vi "Controle_Manip_Main_GUI_Backup2.vi"() -> ()   [LabVIEW 2019] (continued)
                                n1251 = local write "PH_Settings_Params"(w1611) -> ()
                                }
                                frame #2 {
                                n1252 = local read "Spectrum End Wavelength (nm)"() -> (w1629:dbl)
                                n1253 = local read "Spectrum Step Wavelength (nm)"() -> (w1627:dbl)
                                n1254 = local read "Spectrum Start Wavelength (nm)"() -> (w1626:dbl)
                                n1255 = Subtract(x=w1629, y=w1626) -> (x-y=w1631:dbl)
                                n1256 = Divide(x=w1631, y=w1627) -> (x/y=w1630:dbl)
                                n1257 = Increment(x=w1630) -> (x+1=w1628:dbl)
                                n1258 = for {
                                N: w1628 -> [_]
                                tunnel: w1627 -> [w1634]
                                tunnel: w1626 -> [w1635]
                                shift-right: [w1636] -> w1622
                                shift-left: dbl[] [] -> [w1638]
                                shift-right: [w1639] -> w1623
                                shift-left: dbl[] [] -> [w1640]
                                i -> [w1644]
                                stop <- w1632 stop-if-true
                                n1259 = Multiply(x=w1644, y=w1634) -> (x*y=w1643:dbl)
                                n1260 = Add(x=w1635, y=w1643) -> (x+y=w1633:dbl)
                                n1261 = local read "ESP300 COM Port"() -> (w1642:refnum<visa-resource-name>)
                                n1262 = stacked-sequence {
                                tunnel: w1633 -> [w1647 _ w1654 _]
                                tunnel: w1642 -> [w1652 _ _ _]
                                tunnel: [_ _ w1661 _] -> w1641
                                tunnel: w1640 -> [w1650 _ _ _]
                                tunnel: [w1649 _ _ _] -> w1639
                                tunnel: [_ _ _ w1679] -> w1632
                                frame #0 {
                                w1645 = u16 1 items=["Detection"=1, "Excitation"=2] ("HR mode")
                                n1263 = call "MotorWL2Pos.vi"("Mono2 Center WL"=w1647, "HR mode"=w1645) -> ("Mono2 Position"=w1648:dbl)
                                n1264 = control-ref of="Mono2 Wavelength (nm)"() -> (w1646:refnum<vi>)
                                n1265 = control-ref of="Mono2 Motor Pos"() -> (w1651:refnum<vi>)
                                n1266 = call "subVI_Mono2Go2Posv2.vi"("Mono2 Motor Pos"=w1651, "Mono2 Wavelength (nm)"=w1646, "HR mode"=w1645, "Postion (Unit)"=w1648, "ESP300 COM Port"=w1652) -> ()  [unwired: 2 out]
                                n1267 = Insert Into Array(array=w1650, new element=w1647) -> (w1649:dbl[])  [unwired: 1 in]
                                }
                                frame #1 {
                                n1268 = Wait (ms)(milliseconds to wait=u32 20) -> ()  [unwired: 1 out]
                                }
                                frame #2 {
                                n1269 = local read "Photodiode error out"() -> (w1655:errorcluster)
                                n1270 = local read "Photodiode handle out"() -> (w1658:refnum<visa-resource-name>)
                                n1271 = Tick Count (ms)() -> (millisecond timer value=w1664:u32)
                                n1272 = call <instrlib>:"TLPM Set Wavelength.vi"("error in (no error)"=w1655, "Wavelength (0.0)"=w1654, "instrument handle"=w1658) -> ("error out"=w1656:errorcluster, "instrument handle out"=w1657:refnum<visa-resource-name>)  [unwired: 7 in]
                                n1273 = while {
                                shift-right: [w1674] -> w1659
                                shift-left: w1657 -> [w1677]
                                shift-right: [w1675] -> w1660
                                shift-left: w1656 -> [w1676]
                                tunnel: w1664 -> [w1672]
                                shift-right: [w1666] -> w1663
                                shift-left: dbl[] [] -> [w1667]
                                stop <- w1669 stop-if-true
                                n1274 = Tick Count (ms)() -> (millisecond timer value=w1673:u32)
                                n1275 = control-ref of="Excitation Power (uW)"() -> (w1665:refnum<vi>)
                                n1276 = local read "Acq Time (ms)"() -> (w1670:dbl)
                                n1277 = Subtract(x=w1673, y=w1672) -> (x-y=w1671:u32)
                                n1278 = call <instrlib>:"TLPM Measure Power.vi"("error in (no error)"=w1676, "instrument handle"=w1677) -> ("error out"=w1675:errorcluster, "Power"=w1668:dbl, "instrument handle out"=w1674:refnum<visa-resource-name>)  [unwired: 7 in]
                                n1279 = property class="DigNum (strict)"(reference=w1665, "Value"=w1668) -> ()  [unwired: 1 in, 2 out]
                                n1280 = Insert Into Array(array=w1667, new element=w1668) -> (w1666:dbl[])  [unwired: 1 in]
                                n1281 = Greater?(x=w1671, y=w1670) -> (0:w1669:bool)
                                }
                                n1282 = local write "Photodiode handle out"(w1659) -> ()
                                n1283 = local write "Photodiode error out"(w1660) -> ()
                                n1284 = call-poly <vilib>:"Mean.vi"("X"=w1663) -> ("mean"=w1661:dbl)  [unwired: 1 out]
                                }
                                frame #3 {
                                n1285 = control-ref of="MasterStop"() -> (w1678:refnum<vi>)
                                n1286 = control-ref of="Stop Spectrum Custom"() -> ()  [unwired: 1 out]
                                n1287 = property class="Bool (strict)"(reference=w1678) -> ("Value"=w1679:bool)  [unwired: 1 in, 2 out]
                                }
                                }
                                n1288 = Insert Into Array(array=w1638, new element=w1641) -> (w1636:dbl[])  [unwired: 1 in]
                                n1289 = Bundle(w1639, w1636) -> (w1637:cluster{dbl[], dbl[]})  [unwired: 1 in]
                                n1290 = property on="CCD 1D Spectrum Main" class="XYGraph (strict)"("Value"=w1637) -> ()  [unwired: 2 in, 2 out]
                                }
                                n1291 = local write "Data PL Custom Diode Spectrum"(w1622) -> ()
                                n1292 = local write "Wavelength calibration"(w1623) -> ()
                                }
                                frame #3 {
                                n1293 = property on="Elapsed (s)" class="DigNum (strict)"("Visible"=FALSE) -> ()  [unwired: 2 in, 2 out]
                                n1294 = control-ref of="Shutter Ctrls"() -> (w1682:refnum<vi>)
                                n1295 = local read "KCube Shutter On?"() -> (w1681:bool)
                                n1296 = control-ref of="KCube Shutter Device Reference"() -> (w1683:refnum<vi>)
                                n1297 = call "Shutter.vi"("KCube Shutter Device Reference 2"=w1683, "Shutter Ctrls 2"=w1682, "Shutter on?"=w1681) -> ()
                                }
                                }
                              }
                            }
                          }
                          frame #3 {
                            n1298 = property on="Save Custom Diode Spectrum" class="Bool (strict)"("Visible"=TRUE) -> ()  [unwired: 2 in, 2 out]
                            n1299 = control-ref of="MasterPause"() -> (w1685:refnum<vi>)
                            n1300 = control-ref of="MasterStop"() -> (w1687:refnum<vi>)
                            n1301 = local read "Scan Spectrum Cust Params"() -> (w1691:refnum<vi>[])
                            n1302 = property on="Acquire Custom Diode Spectrum" class="Bool (strict)"("Value"=FALSE ("Acquire Custom Diode Spectrum")) -> ()  [unwired: 2 in, 2 out]
                            n1303 = control-ref of="ExperimentStopped?"() -> (w1686:refnum<vi>)
                            n1304 = call "CheckStopAndReset.vi"("ExperimentStopped?"=w1686, "MasterStop"=w1687, "MasterPause"=w1685) -> ()
                            n1305 = call "Enable&Disable_Controls.vi"("Enum"=enum16{"Enabled", "Disabled", "Disabled&Grayed"}."Enabled", "References"=w1691) -> ()  [unwired: 1 in]
                            n1306 = local write "Background taken?"(FALSE ("Background taken?")) -> ()
                          }
                        }
                      }
                      frame "Acquire PLE" {
                        n1307 = stacked-sequence {
                          frame #0 {
                            # "background"
                            n1308 = local read "Background taken?"() -> (w1692:bool)
                            n1309 = case shown="False" w1692 {
                              frame False {
                                n1310 = stacked-sequence {
                                tunnel: [_ _ w1738] -> w1693
                                frame #0 {
                                n1311 = property on="CCD 1D Spectrum Main" class="XYGraph (strict)"("YScale.Offset"=0.0 ("Y Scale.Offset and Multiplier:Offset")) -> ()  [unwired: 2 in, 2 out]
                                }
                                frame #1 {
                                # "make sure shutter is closed"
                                n1312 = local read "KCube Shutter On?"() -> (w1724:bool)
                                n1313 = control-ref of="Shutter Ctrls"() -> (w1728:refnum<vi>)
                                n1314 = property class="Ring (strict)"(reference=w1728) -> ("Value"=w1727:u16)  [unwired: 1 in, 2 out]
                                n1315 = control-ref of="KCube Shutter Device Reference"() -> (w1729:refnum<vi>)
                                n1316 = Equal?(x=w1727, y=u16 0) -> (x = y?=w1725:bool)
                                n1317 = case shown="False" w1725 {
                                tunnel: w1729 -> [w1732 _]
                                tunnel: w1728 -> [w1731 _]
                                tunnel: w1724 -> [w1730 _]
                                frame False {
                                n1318 = call "Shutter.vi"("KCube Shutter Device Reference 2"=w1732, "Shutter Ctrls 2"=w1731, "Shutter on?"=w1730) -> ()
                                }
                                frame True {
                                }
                                }
                                }
                                frame #2 {
                                # "acquire"
                                n1319 = local read "LightField Automation error out"() -> (w1736:errorcluster)
                                n1320 = local read "LightField Automation out"() -> (w1737:refnum<class "LightField Automation.lvclass">)
                                n1321 = local read "Accumulations"() -> (w1733:dbl)
                                n1322 = call "LFA_Capture.vi"("error in (no error)"=w1736, "Frames"=w1733, "LightField Automation in"=w1737) -> ("error out"=w1735:errorcluster, "Data"=w1738:T26, "LightField Automation out"=w1734:refnum<class "LightField Automation.lvclass">)  [unwired: 6 in]
                                n1323 = local write "LightField Automation error out"(w1735) -> ()
                                n1324 = local write "LightField Automation out"(w1734) -> ()
                                }
                                }
                                n1325 = local read "Acq Mode"() -> (w1694:T3)
                                n1326 = case shown="\"Spectrum\", Default" w1694 {
                                selector: w1694 -> [w1695 w1713]
                                tunnel: w1693 -> [w1696 w1714]
                                frame "Spectrum", Default {
                                n1327 = stacked-sequence {
                                tunnel: w1696 -> [_ w1707 _ _]
                                tunnel: w1695 -> [_ w1705 _ _]
                                frame #0 {
                                n1328 = property on="CCD 2D Image Main" class="IntGraph (strict)"("Visible"=FALSE) -> ()  [unwired: 2 in, 2 out]
                                n1329 = property on="CCD 1D Spectrum Main" class="XYGraph (strict)"("Visible"=TRUE) -> ()  [unwired: 2 in, 2 out]
                                }
                                frame #1 {
                                n1330 = local read "Wavelength calibration"() -> (w1704:dbl[])
                                n1331 = local read "CCD ROI"() -> (w1700:T20)
                                n1332 = Divide(x=1239.842, y=w1704) -> (x/y=w1702:dbl[])
                                n1333 = call "PrepareData4Graph.vi"("Wavelength nm"=w1702, "DataLF"=w1707, "CCD ROI"=w1700, "AcqMode"=w1705, "Data type"=T30."Spectre") -> ("Spectrum"=w1706:cluster{"Array 2":dbl[], "Array":dbl[]}, "PLInt out"=w1699:dbl[])  [unwired: 2 in, 2 out]
                                n1334 = local write "CCD 1D Spectrum Main"(w1706) -> ()
                                n1335 = local write "BackgroundSpec"(w1699) -> ()
                                }
                                frame #2 {
                                n1336 = local read "BackgroundSpec"() -> (w1708:dbl[])
                                n1337 = call-poly <vilib>:"Mean.vi"("X"=w1708) -> ("mean"=w1710:dbl)  [unwired: 1 out]
                                n1338 = Negate(x=w1710) -> (-x=w1709:dbl)
                                n1339 = property on="CCD 1D Spectrum Main" class="XYGraph (strict)"("YScale.Offset"=w1709) -> ()  [unwired: 2 in, 2 out]
                                }
                                frame #3 {
                                n1340 = local write "Background taken?"(TRUE ("Background taken?")) -> ()
                                n1341 = property on="Background substract" class="Enum (strict)"("Value"=enum16{"None", "Shutter"}."None" ("Background substract")) -> ()  [unwired: 2 in, 2 out]
                                }
                                }
                                }
                                frame "Image" {
                                n1342 = stacked-sequence {
                                tunnel: w1714 -> [_ w1722]
                                tunnel: w1713 -> [_ w1720]
                                frame #0 {
                                n1343 = property on="CCD 1D Spectrum Main" class="XYGraph (strict)"("Visible"=FALSE) -> ()  [unwired: 2 in, 2 out]
                                n1344 = property on="CCD 2D Image Main" class="IntGraph (strict)"("Visible"=TRUE) -> ()  [unwired: 2 in, 2 out]
                                }
                                frame #1 {
                                n1345 = local read "Wavelength calibration"() -> (w1721:dbl[])
                                n1346 = local read "CCD ROI"() -> (w1717:T20)
                                n1347 = call "PrepareData4Graph.vi"("Wavelength nm"=w1721, "DataLF"=w1722, "CCD ROI"=w1717, "AcqMode"=w1720, "Data type"=T30."Spectre") -> ("Intensity Graph"=w1719:dbl[][])  [unwired: 2 in, 3 out]
                                n1348 = local write "CCD 2D Image Main"(w1719) -> ()
                                }
                                }
                                }
                                }
                              }
                              frame True {
                              }
                            }
                          }
                          frame #1 {
                            # "prep"
                            n1349 = control-ref of="MasterStop"() -> (w1758:refnum<vi>)
                            n1350 = control-ref of="MasterPause"() -> (w1755:refnum<vi>)
                            n1351 = local read "Spectrum Custom Mode"() -> (w1762:u16)
                            n1352 = local read "KCube Shutter On?"() -> (w1761:bool)
                            n1353 = local read "PLE Step (nm)"() -> (w1740:dbl)
                            n1354 = local read "PLE End (nm)"() -> (w1749:dbl)
                            n1355 = local read "Acq Time (ms)"() -> (w1760:dbl)
                            n1356 = local read "PLE Start (nm)"() -> (w1748:dbl)
                            n1357 = property class="Bool (strict)"(reference=w1758, "Visible"=TRUE) -> ()  [unwired: 1 in, 2 out]
                            n1358 = property class="Bool (strict)"(reference=w1755, "Visible"=TRUE) -> ()  [unwired: 1 in, 2 out]
                            n1359 = Bundle("Acq Time (ms)"=w1760, "PLE Start (nm)"=w1748, "PLE Step (nm)"=w1740, "PLE End (nm)"=w1749, "Spectrum Custom Mode"=w1762, "KCube Shutter On?"=w1761) -> (→"Scan PLE":T34)  [unwired: 1 in]
                            n1360 = control-ref of="PLE # Pts"() -> (w1746:refnum<vi>)
                            n1361 = Max & Min(x=w1748, y=w1749) -> (max(x,y)=w1744:dbl, min(x,y)=w1739:dbl)
                            n1362 = local read "Scan PLE AllParams"() -> (w1747:refnum<vi>[])
                            n1363 = property on="Experiment Graph Controls" class="TabCtl (strict)"("Value"=T25."PLE" ("Experiment Graph Controls")) -> ()  [unwired: 2 in, 2 out]
                            n1364 = Build Array (concatenate)(w1747, w1746) -> (w1745:refnum<vi>[])
                            n1365 = control-ref of="Elapsed (s)"() -> (w1753:refnum<vi>)
                            n1366 = property class="DigNum (strict)"(reference=w1753, "Visible"=TRUE) -> ()  [unwired: 1 in, 2 out]
                            n1367 = call "Enable&Disable_Controls.vi"("Enum"=enum16{"Enabled", "Disabled", "Disabled&Grayed"}."Disabled&Grayed", "References"=w1745) -> ()  [unwired: 1 in]
                            n1368 = Add(x=w1744, y=w1740) -> (x+y=w1741:dbl)
                            n1369 = Add(x=w1744, y=w1740) -> (x+y=w1743:dbl)
                            n1370 = property on="PLE Normalised Intensity" class="IntGraph (strict)"("XScale.Multiplier"=w1740, "XScale.Offset"=w1739, "YScale.Maximum"=1340.0 ("Y Scale.Range:Maximum"), "XScale.Minimum"=w1739, "XScale.Maximum"=w1743) -> ()  [unwired: 2 in, 2 out]
                            n1371 = property on="PLE Raw Intensity" class="IntGraph (strict)"("XScale.Multiplier"=w1740, "XScale.Offset"=w1739, "YScale.Maximum"=1340.0 ("Y Scale.Range:Maximum"), "XScale.Minimum"=w1739, "XScale.Maximum"=w1743) -> ()  [unwired: 2 in, 2 out]
                            n1372 = property on="PLE Laser Excitation Power" class="WFGraph (strict)"("XScale.Multiplier"=w1740, "XScale.Offset"=w1739, "XScale.Minimum"=w1739, "XScale.Maximum"=w1741) -> ()  [unwired: 2 in, 2 out]
                            n1373 = property on="PLE Integrated emission efficiency" class="WFGraph (strict)"("XScale.Multiplier"=w1740, "XScale.Offset"=w1739, "XScale.Minimum"=w1739, "XScale.Maximum"=w1741) -> ()  [unwired: 2 in, 2 out]
                          }
                          frame #2 {
                            n1374 = local read "Scan PLE"() -> (w1782:T1)
                            n1375 = Unbundle By Name(w1782) -> ("Acq Time (ms)"=w1775:dbl, "PLE start (nm)"=w1776:dbl, "PLE step (nm)"=w1777:dbl, "PLE end (nm)"=w1781:dbl)  [unwired: 2 out]
                            n1376 = Subtract(x=w1781, y=w1776) -> (x-y=w1780:dbl)
                            n1377 = Get Date/Time In Seconds() -> (seconds since 1Jan1904=w1771:timestamp)
                            n1378 = Divide(x=w1780, y=w1777) -> (x/y=w1779:dbl)
                            n1379 = Increment(x=w1779) -> (x+1=w1778:dbl)
                            n1380 = for {
                              N: w1778 -> [w1788]
                              tunnel: w1777 -> [w1804]
                              tunnel: w1776 -> [w1802]
                              tunnel: w1775 -> [w1800]
                              shift-right: [w1798] -> w1764
                              shift-left: dbl[] [] -> [w1799]
                              shift-right: [w1796] -> w1768
                              shift-left: i32[][] [] -> [w1797]
                              shift-right: [w1794] -> w1767
                              shift-left: dbl[][] [] -> [w1795]
                              tunnel: w1771 -> [w1790]
                              shift-right: [w1786] -> w1769
                              shift-left: dbl[] [] -> [w1787]
                              shift-right: [w1784] -> w1765
                              shift-left: dbl[] [] -> [w1785]
                              i -> [w1793]
                              stop <- w1805 stop-if-true
                              n1381 = Multiply(x=w1793, y=w1804) -> (x*y=w1803:dbl)
                              n1382 = Add(x=w1802, y=w1803) -> (x+y=w1801:dbl)
                              n1383 = Increment(x=w1793) -> (x+1=w1789:i32)
                              n1384 = Divide(x=w1789, y=w1788) -> (x/y=w1783:dbl)
                              n1385 = stacked-sequence {
                                tunnel: w1801 -> [_ w1819 _ _ w1831 _ _ _]
                                tunnel: w1800 -> [_ _ _ _ _ _ _ _]
                                tunnel: w1799 -> [_ _ _ _ w1828 _ _ _]
                                tunnel: [_ _ _ _ w1827 _ _ _] -> w1798
                                tunnel: w1797 -> [_ _ _ _ _ w1861 _ _]
                                tunnel: [_ _ _ _ _ w1860 _ _] -> w1796
                                tunnel: w1795 -> [_ _ _ _ _ w1859 _ _]
                                tunnel: [_ _ _ _ _ w1858 _ _] -> w1794
                                tunnel: w1790 -> [w1812 _ _ _ _ _ _ _]
                                tunnel: w1789 -> [w1811 _ _ _ _ _ _ _]
                                tunnel: w1788 -> [w1810 _ _ _ _ _ _ _]
                                tunnel: w1787 -> [_ _ _ _ _ w1857 _ _]
                                tunnel: [_ _ _ _ _ w1856 _ _] -> w1786
                                tunnel: w1785 -> [_ w1818 _ _ _ _ _ _]
                                tunnel: [_ w1817 _ _ _ _ _ _] -> w1784
                                tunnel: w1783 -> [_ _ w1824 _ _ _ _ _]
                                frame #0 {
                                # "prep"
                                n1386 = control-ref of="Expected (s)"() -> (w1808:refnum<vi>)
                                n1387 = call "Expectedtime.vi"("N"=w1810, "I"=w1811, "Reference time"=w1812) -> ("Expected time"=w1807:dbl, "Elapsed time"=w1809:dbl)
                                n1388 = property on="Elapsed (s)" class="DigNum (strict)"("Value"=w1809) -> ()  [unwired: 2 in, 2 out]
                                n1389 = property class="DigNum (strict)"(reference=w1808, "Value"=w1807) -> ()  [unwired: 1 in, 2 out]
                                }
                                frame #1 {
                                # "move filter to WL and get real wavelength"
                                n1390 = local read "LLTFDevice Interface"() -> (w1820:refnum<k7>)
                                n1391 = control-ref of="Laser on?"() -> (w1821:refnum<vi>)
                                n1392 = call "testmove.vi"("p_TargetWavelength"=w1819, "reference"=w1820) -> ("CurrentWavelength"=w1813:dbl, "CurrentAngle"=w1814:dbl, "Device reference out"=w1815:refnum<k7>, "Device moved"=w1816:bool)  [unwired: 4 in, 2 out]
                                n1393 = local write "CurrentAngle"(w1814) -> ()
                                n1394 = call "ExcWL2LaserrColor.vi"("Wavelength (380 - 780)"=w1819, "Laser on?"=w1821) -> ()  [unwired: 1 in]
                                n1395 = local write "CurrentWL"(w1813) -> ()
                                n1396 = local write "Device moved"(w1816) -> ()
                                n1397 = local write "LLTFDevice Interface"(w1815) -> ()
                                n1398 = Insert Into Array(array=w1818, new element=w1813) -> (w1817:dbl[])  [unwired: 1 in]
                                }
                                frame #2 {
                                # "move microscope objective to focus exc spot"
                                n1399 = local read "KCubePiezoDevice Z Reference"() -> (w1825:refnum<k24>)
                                n1400 = Multiply(x=w1824, y="FocalShift (V KCube)") -> (x*y=w1822:dbl)
                                n1401 = invoke class="KCubePiezo" method="SetOutputVoltage"(reference=w1825, "volts"=w1822) -> ()  [unwired: 2 in, 4 out]
                                }
                                frame #3 {
                                n1402 = Wait (ms)(milliseconds to wait=u32 50) -> ()  [unwired: 1 out]
                                }
                                frame #4 {
                                # "set excwl and measure power"
                                n1403 = local write "Excitation Wavelength (nm)"(w1831) -> ()
                                n1404 = local read "Photodiode Status"() -> (w1829:bool)
                                n1405 = case shown="True" w1829 {
                                tunnel: w1831 -> [_ w1838]
                                tunnel: w1828 -> [w1834 w1837]
                                tunnel: [w1832 w1836] -> w1827
                                frame False {
                                n1406 = Insert Into Array(array=w1834, new element=nan) -> (w1832:dbl[])  [unwired: 1 in]
                                }
                                frame True {
                                n1407 = local read "Photodiode handle out"() -> (w1844:refnum<visa-resource-name>)
                                n1408 = local read "Photodiode error out"() -> (w1843:errorcluster)
                                n1409 = call <instrlib>:"TLPM Set Wavelength.vi"("error in (no error)"=w1843, "Wavelength (0.0)"=w1838, "instrument handle"=w1844) -> ("error out"=w1842:errorcluster, "instrument handle out"=w1841:refnum<visa-resource-name>)  [unwired: 7 in]
                                n1410 = call <instrlib>:"TLPM Measure Power.vi"("error in (no error)"=w1842, "instrument handle"=w1841) -> ("error out"=w1839:errorcluster, "Power"=w1835:dbl, "instrument handle out"=w1840:refnum<visa-resource-name>)  [unwired: 7 in]
                                n1411 = local write "Photodiode handle out"(w1840) -> ()
                                n1412 = local write "Photodiode error out"(w1839) -> ()
                                n1413 = local write "Excitation Power (uW)"(w1835) -> ()
                                n1414 = Insert Into Array(array=w1837, new element=w1835) -> (w1836:dbl[])  [unwired: 1 in]
                                }
                                }
                                "PLE Laser Excitation Power" <- w1827
                                n1415 = control-ref of="Laser on?"() -> (w1830:refnum<vi>)
                                n1416 = call "ExcWL2LaserrColor.vi"("Wavelength (380 - 780)"=w1831, "Laser on?"=w1830) -> ()  [unwired: 1 in]
                                }
                                frame #5 {
                                # "acquire"
                                n1417 = stacked-sequence {
                                tunnel: [_ _ _ w1884] -> w1849
                                tunnel: [_ _ _ w1883] -> w1850
                                frame #0 {
                                # "open shutter if closed"
                                n1418 = control-ref of="KCube Shutter Device Reference"() -> (w1864:refnum<vi>)
                                n1419 = control-ref of="Shutter Ctrls"() -> (w1863:refnum<vi>)
                                n1420 = local read "KCube Shutter On?"() -> (w1862:bool)
                                n1421 = property class="Ring (strict)"(reference=w1863) -> ("Value"=w1865:u16)  [unwired: 1 in, 2 out]
                                n1422 = Equal?(x=w1865, y=u16 0) -> (x = y?=w1867:bool)
                                n1423 = case shown="True" w1867 {
                                tunnel: w1864 -> [_ w1870]
                                tunnel: w1863 -> [_ w1869]
                                tunnel: w1862 -> [_ w1868]
                                frame False {
                                }
                                frame True {
                                n1424 = call "Shutter.vi"("KCube Shutter Device Reference 2"=w1870, "Shutter Ctrls 2"=w1869, "Shutter on?"=w1868) -> ()
                                }
                                }
                                }
                                frame #1 {
                                # "set CCD ROI and acquire"
                                n1425 = local read "LightField Automation error out"() -> (w1879:errorcluster)
                                n1426 = local read "LightField Automation out"() -> (w1871:refnum<class "LightField Automation.lvclass">)
                                n1427 = local read "CCD ROI"() -> (w1878:T20)
                                n1428 = local read "Accumulations"() -> (w1875:dbl)
                                n1429 = call "Adv_SetROI.vi"("error in (no error)"=w1879, "ROI"=w1878, "LightField Automation in"=w1871) -> ("error out"=w1876:errorcluster, "LightField Automation out"=w1877:refnum<class "LightField Automation.lvclass">)  [unwired: 7 in]
                                n1430 = call "LFA_Capture.vi"("error in (no error)"=w1876, "Frames"=w1875, "LightField Automation in"=w1877) -> ("error out"=w1874:errorcluster, "Data"=w1873:T26, "LightField Automation out"=w1872:refnum<class "LightField Automation.lvclass">)  [unwired: 6 in]
                                n1431 = local write "LightField Automation error out"(w1874) -> ()
                                n1432 = local write "LightField Automation out"(w1872) -> ()
                                n1433 = local write "Data"(w1873) -> ()
                                }
                                frame #2 {
                                # "close shutter"
                                n1434 = local read "KCube Shutter On?"() -> (w1882:bool)
                                n1435 = control-ref of="KCube Shutter Device Reference"() -> (w1881:refnum<vi>)
                                n1436 = control-ref of="Shutter Ctrls"() -> (w1880:refnum<vi>)
                                n1437 = call "Shutter.vi"("KCube Shutter Device Reference 2"=w1881, "Shutter Ctrls 2"=w1880, "Shutter on?"=w1882) -> ()
                                }
                                frame #3 {
                                # "Show data accordingly"
                                n1438 = local read "Data"() -> (w1885:T26)
                                n1439 = local read "Acq Mode"() -> (w1886:T3)
                                n1440 = case shown="\"Spectrum\", Default" w1886 {
                                selector: w1886 -> [w1889 w1907]
                                tunnel: w1885 -> [w1890 w1908]
                                tunnel: [w1888 w1906] -> w1884
                                tunnel: [w1887 w1905] -> w1883
                                frame "Spectrum", Default {
                                n1441 = stacked-sequence {
                                tunnel: w1890 -> [_ w1904 _]
                                tunnel: w1889 -> [_ w1903 _]
                                tunnel: [_ w1893 _] -> w1888
                                tunnel: [_ w1892 _] -> w1887
                                frame #0 {
                                }
                                frame #1 {
                                w1891 = u16 4 items=["Sum", "Max", "Sum/s", "Max/s", "Efficiency"] ("Display Mode")
                                n1442 = local read "Excitation Power (uW)"() -> (w1895:dbl)
                                n1443 = local read "Wavelength calibration"() -> (w1902:dbl[])
                                n1444 = local read "CCD ROI"() -> (w1898:T20)
                                n1445 = local read "BackgroundSpec"() -> (w1894:dbl[])
                                n1446 = local read "Acq Time (ms)"() -> (w1896:dbl)
                                n1447 = Divide(x=1239.842, y=w1902) -> (x/y=w1900:dbl[])
                                n1448 = call "PrepareData4Graph.vi"("Wavelength nm"=w1900, "DataLF"=w1904, "CCD ROI"=w1898, "AcqMode"=w1903, "Data type"=T30."Spectre") -> ("PLInt out"=w1893:dbl[])  [unwired: 2 in, 3 out]
                                n1449 = control-ref of="Cnts"() -> (w1897:refnum<vi>)
                                n1450 = call "2Cnts.vi"("Array Background"=w1894, "Pow W"=w1895, "AcqTime ms"=w1896, "Cnts Ref"=w1897, "Display Mode"=w1891, "Array"=w1893) -> ("Value"=w1892:dbl)
                                }
                                frame #2 {
                                }
                                }
                                }
                                frame "Image" {
                                n1451 = stacked-sequence {
                                tunnel: w1908 -> [_ w1917]
                                tunnel: w1907 -> [_ w1915]
                                tunnel: [_ w1912] -> w1906
                                tunnel: [_ nan] -> w1905
                                frame #0 {
                                n1452 = property on="CCD 1D Spectrum Main" class="XYGraph (strict)"("Visible"=FALSE) -> ()  [unwired: 2 in, 2 out]
                                n1453 = property on="CCD 2D Image Main" class="IntGraph (strict)"("Visible"=TRUE) -> ()  [unwired: 2 in, 2 out]
                                }
                                frame #1 {
                                n1454 = local read "Wavelength calibration"() -> (w1916:dbl[])
                                n1455 = local read "CCD ROI"() -> (w1913:T20)
                                n1456 = call "PrepareData4Graph.vi"("Wavelength nm"=w1916, "DataLF"=w1917, "CCD ROI"=w1913, "AcqMode"=w1915, "Data type"=T30."Spectre") -> ("PLInt out"=w1912:dbl[])  [unwired: 2 in, 3 out]
                                }
                                }
                                }
                                }
                                }
                                }
                                n1457 = Insert Into Array(array=w1861, new element=w1849) -> (w1860:i32[][])  [unwired: 2 in]
                                "PLE Raw Intensity" <- w1860
                                n1458 = local read "Excitation Power (uW)"() -> (w1847:dbl)
                                n1459 = local read "BackgroundSpec"() -> (w1851:dbl[])
                                n1460 = local read "Acq Time (ms)"() -> (w1854:dbl)
                                n1461 = Multiply(x=w1847, y=1000000.0) -> (x*y=w1846:dbl)
                                n1462 = Divide(x=w1849, y=w1846) -> (x/y=w1845:dbl[])
                                n1463 = control-ref of="Cnts"() -> (w1855:refnum<vi>)
                                n1464 = Insert Into Array(array=w1859, new element=w1845) -> (w1858:dbl[][])  [unwired: 2 in]
                                "PLE Normalised Intensity" <- w1858
                                n1465 = control-ref of="Display Mode"() -> (w1853:refnum<vi>)
                                n1466 = property class="Ring (strict)"(reference=w1853) -> ("Value"=w1852:u16)  [unwired: 1 in, 2 out]
                                n1467 = call "2Cnts.vi"("Array Background"=w1851, "Pow W"=w1847, "AcqTime ms"=w1854, "Cnts Ref"=w1855, "Display Mode"=w1852, "Array"=w1849) -> ()  [unwired: 1 out]
                                n1468 = Insert Into Array(array=w1857, new element=w1850) -> (w1856:dbl[])  [unwired: 1 in]
                                "PLE Integrated emission efficiency" <- w1856
                                }
                                frame #6 {
                                # "datamanage"
                                }
                                frame #7 {
                                # "pause"
                                n1469 = while {
                                stop <- w1918 continue-if-true
                                n1470 = Wait (ms)(milliseconds to wait=u32 50) -> ()  [unwired: 1 out]
                                n1471 = local read "MasterPause"() -> (w1918:bool)
                                }
                                }
                              }
                              n1472 = Multiply(x=w1783, y=100.0) -> (x*y=w1791:dbl)
                              n1473 = property on="Scan Main Progess Bar" class="Slide (strict)"("Value"=w1791) -> ()  [unwired: 2 in, 2 out]
                              n1474 = control-ref of="MasterStop"() -> (w1806:refnum<vi>)
                              n1475 = property class="Bool (strict)"(reference=w1806) -> ("Value"=w1805:bool)  [unwired: 1 in, 2 out]
                            }
                            "PLE ExcPow" <- w1764
                            "PLE IntegInten" <- w1769
                            "PLE Raw Int" <- w1768
                            "PLE Norm Int" <- w1767
                            "PLE ExcWL" <- w1765
                            n1476 = Build Array(w1765, w1764) -> (→"PLE 2D ExcWL&Pow":dbl[][])
                          }
                          frame #3 {
                            n1477 = control-ref of="Save PLE"() -> (w1931:refnum<vi>)
                            n1478 = control-ref of="Acquire PLE"() -> (w1930:refnum<vi>)
                            n1479 = local read "Auto< ?"() -> (w1929:bool)
                            n1480 = case shown="False" w1929 {
                              tunnel: [TRUE ("Visible") FALSE ("Visible")] -> w1928
                              frame False {
                              }
                              frame True {
                              }
                            }
                            n1481 = control-ref of="MasterPause"() -> (w1932:refnum<vi>)
                            n1482 = control-ref of="MasterStop"() -> (w1934:refnum<vi>)
                            n1483 = property class="Bool (strict)"(reference=w1930, "Visible"=TRUE, "Value"=FALSE) -> ()  [unwired: 1 in, 2 out]
                            n1484 = property class="Bool (strict)"(reference=w1931, "Visible"=w1928) -> ()  [unwired: 1 in, 2 out]
                            n1485 = local read "Scan PLE AllParams"() -> (w1923:refnum<vi>[])
                            n1486 = control-ref of="ExperimentStopped?"() -> (w1933:refnum<vi>)
                            n1487 = call "CheckStopAndReset.vi"("ExperimentStopped?"=w1933, "MasterStop"=w1934, "MasterPause"=w1932) -> ()
                            n1488 = control-ref of="PLE # Pts"() -> (w1922:refnum<vi>)
                            n1489 = Build Array (concatenate)(w1923, w1922) -> (w1921:refnum<vi>[])
                            n1490 = control-ref of="Elapsed (s)"() -> (w1926:refnum<vi>)
                            n1491 = property class="DigNum (strict)"(reference=w1926, "Visible"=FALSE) -> ()  [unwired: 1 in, 2 out]
                            n1492 = call "Enable&Disable_Controls.vi"("Enum"=enum16{"Enabled", "Disabled", "Disabled&Grayed"}."Enabled", "References"=w1921) -> ()  [unwired: 1 in]
                          }
                        }
                      }
                      frame "Acquire Time Trace" {
                        n1493 = stacked-sequence {
                          frame #0 {
                            # "background"
                            n1494 = local read "Background taken?"() -> (w1937:bool)
                            n1495 = case shown="False" w1937 {
                              frame False {
                                n1496 = stacked-sequence {
                                tunnel: [_ _ w1987] -> w1938
                                frame #0 {
                                n1497 = local read "Log file"() -> (w1972:string)
                                n1498 = property on="CCD 1D Spectrum Main" class="XYGraph (strict)"("YScale.Offset"=0.0 ("Y Scale.Offset and Multiplier:Offset")) -> ()  [unwired: 2 in, 2 out]
                                n1499 = call "Write2LogFile.vi"("Add to log file"="Acquiring background", "Log file before"=w1972, "Checkbox"=FALSE) -> ("Log file after"=w1971:string)
                                n1500 = local write "Log file"(w1971) -> ()
                                }
                                frame #1 {
                                # "make sure shutter is closed"
                                n1501 = local read "KCube Shutter On?"() -> (w1973:bool)
                                n1502 = control-ref of="Shutter Ctrls"() -> (w1977:refnum<vi>)
                                n1503 = property class="Ring (strict)"(reference=w1977) -> ("Value"=w1976:u16)  [unwired: 1 in, 2 out]
                                n1504 = control-ref of="KCube Shutter Device Reference"() -> (w1978:refnum<vi>)
                                n1505 = Equal?(x=w1976, y=u16 0) -> (x = y?=w1974:bool)
                                n1506 = case shown="False" w1974 {
                                tunnel: w1978 -> [w1981 _]
                                tunnel: w1977 -> [w1980 _]
                                tunnel: w1973 -> [w1979 _]
                                frame False {
                                n1507 = call "Shutter.vi"("KCube Shutter Device Reference 2"=w1981, "Shutter Ctrls 2"=w1980, "Shutter on?"=w1979) -> ()
                                }
                                frame True {
                                }
                                }
                                }
                                frame #2 {
                                # "acquire"
                                n1508 = local read "LightField Automation error out"() -> (w1985:errorcluster)
                                n1509 = local read "LightField Automation out"() -> (w1986:refnum<class "LightField Automation.lvclass">)
                                n1510 = local read "Accumulations"() -> (w1982:dbl)
                                n1511 = call "LFA_Capture.vi"("error in (no error)"=w1985, "Frames"=w1982, "LightField Automation in"=w1986) -> ("error out"=w1984:errorcluster, "Data"=w1987:T26, "LightField Automation out"=w1983:refnum<class "LightField Automation.lvclass">)  [unwired: 6 in]
                                n1512 = local write "LightField Automation error out"(w1984) -> ()
                                n1513 = local write "LightField Automation out"(w1983) -> ()
                                }
                                }
                                n1514 = local read "Acq Mode"() -> (w1939:T3)
                                n1515 = case shown="\"Spectrum\", Default" w1939 {
                                selector: w1939 -> [w1940 w1958]
                                tunnel: w1938 -> [w1941 w1959]
                                frame "Spectrum", Default {
                                n1516 = stacked-sequence {
                                tunnel: w1941 -> [_ w1952 _ _]
                                tunnel: w1940 -> [_ w1950 _ _]
                                frame #0 {
                                n1517 = property on="CCD 2D Image Main" class="IntGraph (strict)"("Visible"=FALSE) -> ()  [unwired: 2 in, 2 out]
                                n1518 = property on="CCD 1D Spectrum Main" class="XYGraph (strict)"("Visible"=TRUE) -> ()  [unwired: 2 in, 2 out]
                                }
                                frame #1 {
                                n1519 = local read "Wavelength calibration"() -> (w1949:dbl[])
                                n1520 = local read "CCD ROI"() -> (w1945:T20)
                                n1521 = Divide(x=1239.842, y=w1949) -> (x/y=w1947:dbl[])
                                n1522 = call "PrepareData4Graph.vi"("Wavelength nm"=w1947, "DataLF"=w1952, "CCD ROI"=w1945, "AcqMode"=w1950, "Data type"=T30."Spectre") -> ("Spectrum"=w1951:cluster{"Array 2":dbl[], "Array":dbl[]}, "PLInt out"=w1944:dbl[])  [unwired: 2 in, 2 out]
                                n1523 = local write "CCD 1D Spectrum Main"(w1951) -> ()
                                n1524 = local write "BackgroundSpec"(w1944) -> ()
                                }
                                frame #2 {
                                n1525 = local read "BackgroundSpec"() -> (w1953:dbl[])
                                n1526 = call-poly <vilib>:"Mean.vi"("X"=w1953) -> ("mean"=w1955:dbl)  [unwired: 1 out]
                                n1527 = Negate(x=w1955) -> (-x=w1954:dbl)
                                n1528 = property on="CCD 1D Spectrum Main" class="XYGraph (strict)"("YScale.Offset"=w1954) -> ()  [unwired: 2 in, 2 out]
                                }
                                frame #3 {
                                n1529 = local write "Background taken?"(TRUE ("Background taken?")) -> ()
                                n1530 = property on="Background substract" class="Enum (strict)"("Value"=enum16{"None", "Shutter"}."None" ("Background substract")) -> ()  [unwired: 2 in, 2 out]
                                }
                                }
                                }
                                frame "Image" {
                                n1531 = stacked-sequence {
                                tunnel: w1959 -> [_ w1967]
                                tunnel: w1958 -> [_ w1965]
                                frame #0 {
                                n1532 = property on="CCD 1D Spectrum Main" class="XYGraph (strict)"("Visible"=FALSE) -> ()  [unwired: 2 in, 2 out]
                                n1533 = property on="CCD 2D Image Main" class="IntGraph (strict)"("Visible"=TRUE) -> ()  [unwired: 2 in, 2 out]
                                }
                                frame #1 {
                                n1534 = local read "Wavelength calibration"() -> (w1966:dbl[])
                                n1535 = local read "CCD ROI"() -> (w1962:T20)
                                n1536 = call "PrepareData4Graph.vi"("Wavelength nm"=w1966, "DataLF"=w1967, "CCD ROI"=w1962, "AcqMode"=w1965, "Data type"=T30."Spectre") -> ("Intensity Graph"=w1964:dbl[][])  [unwired: 2 in, 3 out]
                                n1537 = local write "CCD 2D Image Main"(w1964) -> ()
                                }
                                }
                                }
                                }
                              }
                              frame True {
                              }
                            }
                          }
                          frame #1 {
                            # "measurement"
                            n1538 = stacked-sequence {
                              frame #0 {
                                w1988 = FALSE ("Visible")
                                # "open shutter once"
                                n1539 = local read "KCube Shutter On?"() -> (w1989:bool)
                                n1540 = control-ref of="Shutter Ctrls"() -> (w1991:refnum<vi>)
                                n1541 = control-ref of="KCube Shutter Device Reference"() -> (w1990:refnum<vi>)
                                n1542 = call "Shutter.vi"("KCube Shutter Device Reference 2"=w1990, "Shutter Ctrls 2"=w1991, "Shutter on?"=w1989) -> ()
                                n1543 = property on="Acquire Time Trace" class="Bool (strict)"("Visible"=w1988) -> ()  [unwired: 2 in, 2 out]
                                n1544 = property on="Save Spectrum N" class="Bool (strict)"("Visible"=w1988) -> ()  [unwired: 2 in, 2 out]
                              }
                              frame #1 {
                                # "acquire N spectra"
                                n1545 = local read "CCD ROI"() -> (w1992:T20)
                                n1546 = local read "Acquire N: N"() -> (w1999:dbl)
                                n1547 = local read "LightField Automation error out"() -> (w1996:errorcluster)
                                n1548 = local read "LightField Automation out"() -> (w1995:refnum<class "LightField Automation.lvclass">)
                                n1549 = local read "Acq Mode"() -> (w1998:T3)
                                n1550 = call "LFA_Capture.vi"("error in (no error)"=w1996, "Frames"=w1999, "LightField Automation in"=w1995) -> ("error out"=w1993:errorcluster, "Data"=w1997:T26, "LightField Automation out"=w1994:refnum<class "LightField Automation.lvclass">)  [unwired: 6 in]
                                n1551 = case shown="\"Image\"" w1998 {
                                selector: w1998 -> [w2004 w2014]
                                tunnel: w1997 -> [w2006 w2015]
                                tunnel: w1992 -> [w2002 w2012]
                                frame "Spectrum", Default {
                                n1552 = local read "Wavelength calibration"() -> (w2005:dbl[])
                                n1553 = call "PrepareData4Graph.vi"("Wavelength nm"=w2005, "DataLF"=w2006, "CCD ROI"=w2002, "AcqMode"=w2004, "Data type"=T30."Time Trace") -> ("Intensity Graph"=w2001:dbl[][])  [unwired: 2 in, 3 out]
                                n1554 = Transpose 2D Array(2D array=w2001) -> (transposed array=w2000:dbl[][])
                                n1555 = local write "CCD 2D Image Main"(w2000) -> ()
                                }
                                frame "Image" {
                                n1556 = local read "Wavelength calibration"() -> (w2008:dbl[])
                                n1557 = Divide(x=1239.842, y=w2008) -> (x/y=w2007:dbl[])
                                n1558 = call "PrepareData4Graph.vi"("Wavelength nm"=w2007, "DataLF"=w2015, "CCD ROI"=w2012, "AcqMode"=w2014, "Data type"=T30."Time Trace") -> ("Intensity Graph"=w2011:dbl[][])  [unwired: 2 in, 3 out]
                                n1559 = Transpose 2D Array(2D array=w2011) -> (transposed array=w2010:dbl[][])
                                n1560 = local write "CCD 2D Image Main"(w2010) -> ()
                                }
                                }
                                n1561 = local write "LightField Automation error out"(w1993) -> ()
                                n1562 = local write "LightField Automation out"(w1994) -> ()
                                n1563 = local write "Data"(w1997) -> ()
                              }
                              frame #2 {
                                # "close shutter"
                                n1564 = local read "KCube Shutter On?"() -> (w2016:bool)
                                n1565 = control-ref of="Shutter Ctrls"() -> (w2018:refnum<vi>)
                                n1566 = control-ref of="KCube Shutter Device Reference"() -> (w2017:refnum<vi>)
                                n1567 = call "Shutter.vi"("KCube Shutter Device Reference 2"=w2017, "Shutter Ctrls 2"=w2018, "Shutter on?"=w2016) -> ()
                              }
                              frame #3 {
                                # "finish"
                                n1568 = property on="CCD 1D Spectrum Main" class="XYGraph (strict)"("Visible"=FALSE) -> ()  [unwired: 2 in, 2 out]
                                n1569 = property on="CCD 2D Image Main" class="IntGraph (strict)"("Visible"=TRUE) -> ()  [unwired: 2 in, 2 out]
                                n1570 = local read "Auto< ?"() -> (w2020:bool)
                                n1571 = Not(x=w2020) -> (.not. x?=w2021:bool)
                                n1572 = property on="Save Spectrum N" class="Bool (strict)"("Visible"=w2021) -> ()  [unwired: 2 in, 2 out]
                                n1573 = property on="Acquire Time Trace" class="Bool (strict)"("Visible"=TRUE) -> ()  [unwired: 2 in, 2 out]
                              }
                            }
                          }
                        }
                      }
                      frame "Acquire Polarisation" {
                        n1574 = stacked-sequence {
                          frame #0 {
                            # "background"
                            n1575 = local read "Background taken?"() -> (w2024:bool)
                            n1576 = case shown="False" w2024 {
                              frame False {
                                n1577 = stacked-sequence {
                                tunnel: [_ _ w2074] -> w2025
                                frame #0 {
                                n1578 = local read "Log file"() -> (w2059:string)
                                n1579 = property on="CCD 1D Spectrum Main" class="XYGraph (strict)"("YScale.Offset"=0.0 ("Y Scale.Offset and Multiplier:Offset")) -> ()  [unwired: 2 in, 2 out]
                                n1580 = call "Write2LogFile.vi"("Add to log file"="Acquiring background", "Log file before"=w2059, "Checkbox"=FALSE) -> ("Log file after"=w2058:string)
                                n1581 = local write "Log file"(w2058) -> ()
                                }
                                frame #1 {
                                # "make sure shutter is closed"
                                n1582 = local read "KCube Shutter On?"() -> (w2060:bool)
                                n1583 = control-ref of="Shutter Ctrls"() -> (w2064:refnum<vi>)
                                n1584 = property class="Ring (strict)"(reference=w2064) -> ("Value"=w2063:u16)  [unwired: 1 in, 2 out]
                                n1585 = control-ref of="KCube Shutter Device Reference"() -> (w2065:refnum<vi>)
                                n1586 = Equal?(x=w2063, y=u16 0) -> (x = y?=w2061:bool)
                                n1587 = case shown="False" w2061 {
                                tunnel: w2065 -> [w2068 _]
                                tunnel: w2064 -> [w2067 _]
                                tunnel: w2060 -> [w2066 _]
                                frame False {
                                n1588 = call "Shutter.vi"("KCube Shutter Device Reference 2"=w2068, "Shutter Ctrls 2"=w2067, "Shutter on?"=w2066) -> ()
                                }
                                frame True {
                                }
                                }
                                }
                                frame #2 {
                                # "acquire"
                                n1589 = local read "LightField Automation error out"() -> (w2072:errorcluster)
                                n1590 = local read "LightField Automation out"() -> (w2073:refnum<class "LightField Automation.lvclass">)
                                n1591 = local read "Accumulations"() -> (w2069:dbl)
                                n1592 = call "LFA_Capture.vi"("error in (no error)"=w2072, "Frames"=w2069, "LightField Automation in"=w2073) -> ("error out"=w2071:errorcluster, "Data"=w2074:T26, "LightField Automation out"=w2070:refnum<class "LightField Automation.lvclass">)  [unwired: 6 in]
                                n1593 = local write "LightField Automation error out"(w2071) -> ()
                                n1594 = local write "LightField Automation out"(w2070) -> ()
                                }
                                }
                                n1595 = local read "Acq Mode"() -> (w2026:T3)
                                n1596 = case shown="\"Spectrum\", Default" w2026 {
                                selector: w2026 -> [w2027 w2045]
                                tunnel: w2025 -> [w2028 w2046]
                                frame "Spectrum", Default {
                                n1597 = stacked-sequence {
                                tunnel: w2028 -> [_ w2039 _ _]
                                tunnel: w2027 -> [_ w2037 _ _]
                                frame #0 {
                                n1598 = property on="CCD 2D Image Main" class="IntGraph (strict)"("Visible"=FALSE) -> ()  [unwired: 2 in, 2 out]
                                n1599 = property on="CCD 1D Spectrum Main" class="XYGraph (strict)"("Visible"=TRUE) -> ()  [unwired: 2 in, 2 out]
                                }
                                frame #1 {
                                n1600 = local read "Wavelength calibration"() -> (w2036:dbl[])
                                n1601 = local read "CCD ROI"() -> (w2032:T20)
                                n1602 = Divide(x=1239.842, y=w2036) -> (x/y=w2034:dbl[])
                                n1603 = call "PrepareData4Graph.vi"("Wavelength nm"=w2034, "DataLF"=w2039, "CCD ROI"=w2032, "AcqMode"=w2037, "Data type"=T30."Spectre") -> ("Spectrum"=w2038:cluster{"Array 2":dbl[], "Array":dbl[]}, "PLInt out"=w2031:dbl[])  [unwired: 2 in, 2 out]
                                n1604 = local write "CCD 1D Spectrum Main"(w2038) -> ()
                                n1605 = local write "BackgroundSpec"(w2031) -> ()
                                }
                                frame #2 {
                                n1606 = local read "BackgroundSpec"() -> (w2040:dbl[])
                                n1607 = call-poly <vilib>:"Mean.vi"("X"=w2040) -> ("mean"=w2042:dbl)  [unwired: 1 out]
                                n1608 = Negate(x=w2042) -> (-x=w2041:dbl)
                                n1609 = property on="CCD 1D Spectrum Main" class="XYGraph (strict)"("YScale.Offset"=w2041) -> ()  [unwired: 2 in, 2 out]
                                }
                                frame #3 {
                                n1610 = local write "Background taken?"(TRUE ("Background taken?")) -> ()
                                n1611 = property on="Background substract" class="Enum (strict)"("Value"=enum16{"None", "Shutter"}."None" ("Background substract")) -> ()  [unwired: 2 in, 2 out]
                                }
                                }
                                }
                                frame "Image" {
                                n1612 = stacked-sequence {
                                tunnel: w2046 -> [_ w2054]
                                tunnel: w2045 -> [_ w2052]
                                frame #0 {
                                n1613 = property on="CCD 1D Spectrum Main" class="XYGraph (strict)"("Visible"=FALSE) -> ()  [unwired: 2 in, 2 out]
                                n1614 = property on="CCD 2D Image Main" class="IntGraph (strict)"("Visible"=TRUE) -> ()  [unwired: 2 in, 2 out]
                                }
                                frame #1 {
                                n1615 = local read "Wavelength calibration"() -> (w2053:dbl[])
                                n1616 = local read "CCD ROI"() -> (w2049:T20)
                                n1617 = call "PrepareData4Graph.vi"("Wavelength nm"=w2053, "DataLF"=w2054, "CCD ROI"=w2049, "AcqMode"=w2052, "Data type"=T30."Spectre") -> ("Intensity Graph"=w2051:dbl[][])  [unwired: 2 in, 3 out]
                                n1618 = local write "CCD 2D Image Main"(w2051) -> ()
                                }
                                }
                                }
                                }
                              }
                              frame True {
                              }
                            }
                          }
                          frame #1 {